vi "TLB Native Dynamic Events ver 0.26d.vi"() -> ()   [LabVIEW 2018] (continued)
          tunnel: w289 -> [_ _ _ _ _ _ _ _ _ _ _ _ _ _ _ _ _ _ _ _ _ _ _ _ _ _ _ _ _ _ _ _ _ _ _ _ _ _ _ _ _ _ _ _ _ _ _ _ _ _ _ _ _ _ _ _ _ _ _]
          tunnel: w288 -> [_ _ _ _ _ _ _ _ _ _ _ _ _ _ _ _ _ _ _ _ _ _ _ _ _ _ _ _ _ _ _ _ _ _ _ _ _ _ _ _ _ _ _ _ _ _ _ _ _ _ _ _ _ _ _ _ _ _ _]
          tunnel: w287 -> [_ _ _ _ _ _ _ _ _ _ _ _ _ _ _ _ _ _ _ _ _ _ _ _ _ _ _ _ _ _ _ _ _ _ _ _ _ _ _ _ _ _ w2183 _ w2271 _ _ _ _ _ _ _ _ _ _ w2774 _ _ _]
          frame 0 {
            # ">>> yStepper command>>>"
          }
          frame 1 {
            # ">>> yStepper command>>>"
            n215 = for {
              shift-right: [w366] -> w360
              shift-left: w363 -> [w365]
              tunnel: string[] ["INIT", "RESET ARM", "RESET FLAGS", "RESET YAW", "NAVX CALIBRATE"] -> [w364] mode=indexing
              n216 = Enqueue Element(queue=w365, element=w364) -> (queue out=w366:refnum<queue>)  [unwired: 2 in, 2 out]
            }
            n217 = Bundle By Name(cluster=w358, "yStepper desired"=u8 0) -> (w357:T20)
            n218 = Bundle By Name(cluster=w355, "ySpeed"=0.0, "xSpeed"=0.0, "wSpeed"=0.0) -> (w354:T19)
          }
          frame 3 {
            # ">>Action Queue>>"
            # ">>> Motor control cluster >>>"
            # ">>> yStepper command>>>"
            n219 = Flush Queue(queue=w373, error in (no error)=w372) -> ()  [unwired: 3 out]
            n220 = for {
              shift-right: [w379] -> w374
              shift-left: w375 -> [w378]
              tunnel: string[] ["STOP", "RESET ENCODERS", "RESET YAW", "RESET ARM", "RESET ALL SENSORS", "DISPOSE CAM BUFFERS", "DISPOSE PROC BUFFERS", "CAM CLOSE", ""] -> [w377] mode=indexing
              n221 = Enqueue Element(queue=w378, element=w377) -> (queue out=w379:refnum<queue>)  [unwired: 2 in, 2 out]
            }
          }
          frame 4, Default {
            # ">>> Motor control cluster >>>"
            # ">>> yStepper command>>>"
            n222 = Dequeue Element(queue=w391, timeout in ms (-1)=w390, error in (no error)=w386) -> (element=w389:T10)  [unwired: 3 out]
            n223 = case shown="\"Start Task 9\"" w389 {
              tunnel: [w394 w402 w410 w418 w426 w434 w442 w450 w458 w465 w475 w483 w490 w493] -> w385
              tunnel: w388 -> [w395 w403 w411 w419 w427 w435 w443 w451 w459 w466 w474 w482 w490 w494]
              tunnel: [State_Type_Definitions,_for_0.26g_versions_and_later_2."Task 1A" ("Enum") State_Type_Definitions,_for_0.26g_versions_and_later_2."Task 2:Raise Arm" ("Enum") State_Type_Definitions,_for_0.26g_versions_and_later_2."Task 3" ("Enum") State_Type_Definitions,_for_0.26g_versions_and_later_2."Task 4_A" ("Enum") State_Type_Definitions,_for_0.26g_versions_and_later_2."Task 5A" ("Enum") State_Type_Definitions,_for_0.26g_versions_and_later_2."Task 6_A" ("Enum") State_Type_Definitions,_for_0.26g_versions_and_later_2."Task 8A: RAISE ARM" ("Enum") State_Type_Definitions,_for_0.26g_versions_and_later_2."Task 8A: RAISE ARM" ("Enum") State_Type_Definitions,_for_0.26g_versions_and_later_2."Task 8A: RAISE ARM" ("Enum") State_Type_Definitions,_for_0.26g_versions_and_later_2."Task 8A: RAISE ARM" ("Enum") State_Type_Definitions,_for_0.26g_versions_and_later_2."Task 9A: Raise Arm" ("Enum") State_Type_Definitions,_for_0.26g_versions_and_later_2."Task A1: Task 9 Open cam" ("Enum") State_Type_Definitions,_for_0.26g_versions_and_later_2."Idle" ("Enum") State_Type_Definitions,_for_0.26g_versions_and_later_2."Shutdown" ("Enum")] -> w387
              tunnel: [enum16{"Ball", "Soap", "Gel", "Pipe", "None"}."None" ("Object recognition mode") enum16{"Ball", "Soap", "Gel", "Pipe", "None"}."None" ("Object recognition mode") enum16{"Ball", "Soap", "Gel", "Pipe", "None"}."None" ("Object recognition mode") enum16{"Ball", "Soap", "Gel", "Pipe", "None"}."None" ("Object recognition mode") enum16{"Ball", "Soap", "Gel", "Pipe", "None"}."None" ("Object recognition mode") enum16{"Ball", "Soap", "Gel", "Pipe", "None"}."None" ("Object recognition mode") enum16{"Ball", "Soap", "Gel", "Pipe", "None"}."Ball" ("Object recognition mode") enum16{"Ball", "Soap", "Gel", "Pipe", "None"}."Gel" ("Object recognition mode") enum16{"Ball", "Soap", "Gel", "Pipe", "None"}."Pipe" ("Object recognition mode") enum16{"Ball", "Soap", "Gel", "Pipe", "None"}."Soap" ("Object recognition mode") enum16{"Ball", "Soap", "Gel", "Pipe", "None"}."None" ("Object recognition mode") enum16{"Ball", "Soap", "Gel", "Pipe", "None"}."None" ("Object recognition mode") enum16{"Ball", "Soap", "Gel", "Pipe", "None"}."None" ("Object recognition mode") enum16{"Ball", "Soap", "Gel", "Pipe", "None"}."None" ("Object recognition mode")] -> w380
              frame "Start Task 1" {
                n224 = for {
                  shift-right: [w399] -> w394
                  shift-left: w395 -> [w398]
                  tunnel: string[] ["RESET ENCODERS", "RESET YAW", "FORWARD", "READ ENCODERS"] -> [w397] mode=indexing
                  n225 = Enqueue Element(queue=w398, element=w397) -> (queue out=w399:refnum<queue>)  [unwired: 2 in, 2 out]
                }
              }
              frame "Start Task 2" {
                n226 = for {
                  shift-right: [w407] -> w402
                  shift-left: w403 -> [w406]
                  tunnel: string[] ["RESET ENCODERS", "RESET YAW", "READ ULTRASONIC", "ARDUINO - ULTRASONIC"] -> [w405] mode=indexing
                  n227 = Enqueue Element(queue=w406, element=w405) -> (queue out=w407:refnum<queue>)  [unwired: 2 in, 2 out]
                }
              }
              frame "Start Task 3" {
                n228 = for {
                  shift-right: [w415] -> w410
                  shift-left: w411 -> [w414]
                  tunnel: string[] ["RESET ENCODERS", "READ ENCODERS", "R-ACW"] -> [w413] mode=indexing
                  n229 = Enqueue Element(queue=w414, element=w413) -> (queue out=w415:refnum<queue>)  [unwired: 2 in, 2 out]
                }
              }
              frame "Start Task 4" {
                n230 = for {
                  shift-right: [w423] -> w418
                  shift-left: w419 -> [w422]
                  tunnel: string[] ["RESET YAW", "RESET ENCODERS", "RESET ARM", "RESET FLAGS", "", ""] -> [w421] mode=indexing
                  n231 = Enqueue Element(queue=w422, element=w421) -> (queue out=w423:refnum<queue>)  [unwired: 2 in, 2 out]
                }
              }
              frame "Start Task 5" {
                n232 = for {
                  shift-right: [w431] -> w426
                  shift-left: w427 -> [w430]
                  tunnel: string[] ["RESET YAW", "RESET ENCODERS", "RESET ARM", "RESET ALL SENSORS", "", ""] -> [w429] mode=indexing
                  n233 = Enqueue Element(queue=w430, element=w429) -> (queue out=w431:refnum<queue>)  [unwired: 2 in, 2 out]
                }
              }
              frame "Start Task 6" {
                n234 = for {
                  shift-right: [w439] -> w434
                  shift-left: w435 -> [w438]
                  tunnel: string[] ["OPEN LOG CAM ", "", "", "", "", ""] -> [w437] mode=indexing
                  n235 = Enqueue Element(queue=w438, element=w437) -> (queue out=w439:refnum<queue>)  [unwired: 2 in, 2 out]
                }
              }
              frame "Start Task 8 - BALL" {
                n236 = for {
                  shift-right: [w447] -> w442
                  shift-left: w443 -> [w446]
                  tunnel: string[] ["RESET YAW", "RESET ENCODERS", "RESET ARM", "RESET FLAGS"] -> [w445] mode=indexing
                  n237 = Enqueue Element(queue=w446, element=w445) -> (queue out=w447:refnum<queue>)  [unwired: 2 in, 2 out]
                }
              }
              frame "Start Task 8 - Gel" {
                n238 = for {
                  shift-right: [w455] -> w450
                  shift-left: w451 -> [w454]
                  tunnel: string[] ["RESET YAW", "RESET ENCODERS", "RESET ARM", "RESET FLAGS"] -> [w453] mode=indexing
                  n239 = Enqueue Element(queue=w454, element=w453) -> (queue out=w455:refnum<queue>)  [unwired: 2 in, 2 out]
                }
              }
              frame "Start Task 8 - Pipe" {
                n240 = for {
                  shift-right: [w463] -> w458
                  shift-left: w459 -> [w462]
                  tunnel: string[] ["RESET YAW", "RESET ENCODERS", "RESET ARM", "RESET FLAGS"] -> [w461] mode=indexing
                  n241 = Enqueue Element(queue=w462, element=w461) -> (queue out=w463:refnum<queue>)  [unwired: 2 in, 2 out]
                }
              }
              frame "Start Task 8 - Soap" {
                n242 = for {
                  shift-right: [w471] -> w465
                  shift-left: w466 -> [w470]
                  tunnel: string[] ["RESET YAW", "RESET ENCODERS", "RESET ARM", "RESET FLAGS"] -> [w469] mode=indexing
                  n243 = Enqueue Element(queue=w470, element=w469) -> (queue out=w471:refnum<queue>)  [unwired: 2 in, 2 out]
                }
              }
              frame "Start Task 9" {
                n244 = for {
                  shift-right: [w479] -> w475
                  shift-left: w474 -> [w478]
                  tunnel: string[] ["Z STEPPER BOX HEIGHT", "READ STEPPER VALUES", "", ""] -> [w477] mode=indexing
                  n245 = Enqueue Element(queue=w478, element=w477) -> (queue out=w479:refnum<queue>)  [unwired: 2 in, 2 out]
                }
              }
              frame "Start Task A" {
                n246 = for {
                  shift-right: [w487] -> w483
                  shift-left: w482 -> [w486]
                  tunnel: string[] ["RESET ENCODERS", "READ ENCODERS", "RESET YAW", "Z STEPPER BOX HEIGHT"] -> [w485] mode=indexing
                  n247 = Enqueue Element(queue=w486, element=w485) -> (queue out=w487:refnum<queue>)  [unwired: 2 in, 2 out]
                }
              }
              frame "None", Default {
              }
              frame "Exit" {
                n248 = for {
                  shift-right: [w498] -> w493
                  shift-left: w494 -> [w497]
                  tunnel: string[] ["STOP", "RESET ENCODERS", "RESET YAW", "EXIT"] -> [w496] mode=indexing
                  n249 = Enqueue Element(queue=w497, element=w496) -> (queue out=w498:refnum<queue>)  [unwired: 2 in, 2 out]
                }
              }
            }
          }
          frame 5 {
            # ">> Item Selection Bias >>"
            # ">>> yStepper command>>>"
            n250 = for {
              shift-right: [w509] -> w503
              shift-left: w505 -> [w508]
              tunnel: string[] ["INIT", "RESET ENCODERS", "RESET FLAGS", "CAM CLOSE", "DISPOSE BUFFERS", "EXIT", ""] -> [w507] mode=indexing
              n251 = Enqueue Element(queue=w508, element=w507) -> (queue out=w509:refnum<queue>)  [unwired: 2 in, 2 out]
            }
          }
          frame 6 {
            # ">>> Motor control cluster >>>"
            # ">> Line detection >>"
            # ">> Checks if 1 metre moved >>"
            # ">>> yStepper command>>>"
            # "Use 250"
            n252 = Greater?(x=w519, y=265.0) -> (0:w513:bool)
            n253 = Dequeue Element(queue=w526, timeout in ms (-1)=w525, error in (no error)=w524) -> (element=w523:T10)  [unwired: 3 out]
            n254 = And(x=w512, y=w513) -> (x .and. y?=w510:bool)
            n255 = case shown="\"Start Task 1\", Default" w523 {
              tunnel: w511 -> [w527 _]
              tunnel: [w537 State_Type_Definitions,_for_0.26g_versions_and_later_2."True Stop" ("Enum")] -> w522
              tunnel: w521 -> [w535 w552]
              tunnel: [w534 w551] -> w520
              tunnel: [State_Type_Definitions,_for_0.26g_versions_and_later_2."Idle" ("Enum") State_Type_Definitions,_for_0.26g_versions_and_later_2."Shutdown" ("Enum")] -> w517
              tunnel: w510 -> [w528 _]
              frame "Start Task 1", Default {
                n256 = Or(x=w528, y=w527) -> (x .or. y?=w529:bool)
                n257 = case shown="True" w529 {
                  tunnel: w535 -> [w540 w546]
                  tunnel: [w539 w544] -> w534
                  frame False {
                    n258 = for {
                      shift-right: [w542] -> w539
                      shift-left: w540 -> [w543]
                      tunnel: string[] ["READ ENCODERS", "READ NAVX", "FORWARD", "READ LINE SENSOR"] ("element") -> [w541] mode=indexing
                      n259 = Enqueue Element(queue=w543, element=w541) -> (queue out=w542:refnum<queue>)  [unwired: 2 in, 2 out]
                    }
                  }
                  frame True {
                    n260 = for {
                      shift-right: [w548] -> w544
                      shift-left: w546 -> [w549]
                      tunnel: string[] ["RESET YAW", "RESET ENCODERS", "STOP", ""] -> [w547] mode=indexing
                      n261 = Enqueue Element(queue=w549, element=w547) -> (queue out=w548:refnum<queue>)  [unwired: 2 in, 2 out]
                    }
                  }
                }
                n262 = Select(t=State_Type_Definitions,_for_0.26g_versions_and_later_2."True Stop" ("Enum"), s=w527, f=State_Type_Definitions,_for_0.26g_versions_and_later_2."Task 1B" ("Enum")) -> (s? t:f=w532:T18)
                n263 = Select(t=w532, s=w528, f=State_Type_Definitions,_for_0.26g_versions_and_later_2."Task 1A" ("Enum")) -> (s? t:f=w537:T18)
              }
              frame "Exit" {
                n264 = for {
                  shift-right: [w556] -> w551
                  shift-left: w552 -> [w557]
                  tunnel: string[] ["STOP", "RESET ENCODERS", "RESET YAW", ""] -> [w555] mode=indexing
                  n265 = Enqueue Element(queue=w557, element=w555) -> (queue out=w556:refnum<queue>)  [unwired: 2 in, 2 out]
                }
              }
            }
          }
          frame 7 {
            # ">>> Motor control cluster >>>"
            # ">> Line detection >>"
            # ">> Adds small distance overhead after 1M >>"
            # ">>> yStepper command>>>"
            n266 = Greater?(x=w564, y=50.0) -> (0:w558:bool)
            n267 = Dequeue Element(queue=w573, timeout in ms (-1)=w572, error in (no error)=w571) -> (element=w570:T10)  [unwired: 3 out]
            n268 = Or(x=w558, y=w565) -> (x .or. y?=w569:bool)
            n269 = case shown="\"Start Task 1\", Default" w570 {
              tunnel: w569 -> [w576 _]
              tunnel: [w580 State_Type_Definitions,_for_0.26g_versions_and_later_2."True Stop" ("Enum")] -> w568
              tunnel: w567 -> [w577 w595]
              tunnel: [w575 w594] -> w566
              tunnel: [State_Type_Definitions,_for_0.26g_versions_and_later_2."Idle" ("Enum") State_Type_Definitions,_for_0.26g_versions_and_later_2."Shutdown" ("Enum")] -> w562
              frame "Start Task 1", Default {
                n270 = case shown="True" w576 {
                  tunnel: w577 -> [w583 w589]
                  tunnel: [w582 w587] -> w575
                  frame False {
                    n271 = for {
                      shift-right: [w585] -> w582
                      shift-left: w583 -> [w586]
                      tunnel: string[] ["READ ENCODERS", "READ NAVX", "FORWARD", "READ LINE SENSOR"] ("element") -> [w584] mode=indexing
                      n272 = Enqueue Element(queue=w586, element=w584) -> (queue out=w585:refnum<queue>)  [unwired: 2 in, 2 out]
                    }
                  }
                  frame True {
                    n273 = for {
                      shift-right: [w591] -> w587
                      shift-left: w589 -> [w592]
                      tunnel: string[] ["RESET YAW", "RESET ENCODERS", "STOP", ""] -> [w590] mode=indexing
                      n274 = Enqueue Element(queue=w592, element=w590) -> (queue out=w591:refnum<queue>)  [unwired: 2 in, 2 out]
                    }
                  }
                }
                n275 = Select(t=State_Type_Definitions,_for_0.26g_versions_and_later_2."True Stop" ("Enum"), s=w576, f=State_Type_Definitions,_for_0.26g_versions_and_later_2."Task 1B" ("Enum")) -> (s? t:f=w580:T18)
              }
              frame "Exit" {
                n276 = for {
                  shift-right: [w599] -> w594
                  shift-left: w595 -> [w600]
                  tunnel: string[] ["STOP", "RESET ENCODERS", "RESET YAW", ""] -> [w598] mode=indexing
                  n277 = Enqueue Element(queue=w600, element=w598) -> (queue out=w599:refnum<queue>)  [unwired: 2 in, 2 out]
                }
              }
            }
          }
          frame 8 {
            # ">> Stepper height reeached >>"
            # ">>> yStepper command>>>"
            # ">> Manual override >>"
            n278 = Dequeue Element(queue=w606, timeout in ms (-1)=w605, error in (no error)=w604) -> (element=w615:T10)  [unwired: 3 out]
            n279 = Equal?(x=w608, y=u8 60) -> (x = y?=w613:bool)
            n280 = case shown="\"Start Task 1\", Default" w615 {
              tunnel: [w626 State_Type_Definitions,_for_0.26g_versions_and_later_2."True Stop" ("Enum")] -> w610
              tunnel: [w624 w641] -> w603
              tunnel: w612 -> [w623 _]
              tunnel: w611 -> [w617 _]
              tunnel: [State_Type_Definitions,_for_0.26g_versions_and_later_2."Idle" ("Enum") State_Type_Definitions,_for_0.26g_versions_and_later_2."Shutdown" ("Enum")] -> w609
              tunnel: w613 -> [w616 _]
              frame "Start Task 1", Default {
                # ">> WIill proceed to part ii if not manual override >>"
                # ">>If ENABLE or Trigger is set to true>>"
                n281 = Or(x=w616, y=w617) -> (x .or. y?=w618:bool)
                n282 = case shown="True" w616 {
                  tunnel: [w629 w635] -> w624
                  tunnel: w623 -> [w628 w634]
                  frame False {
                    n283 = for {
                      shift-right: [w631] -> w629
                      shift-left: w628 -> [w632]
                      tunnel: string[] ["Z STEPPER CAM HEIGHT", "READ STEPPER VALUES"] ("element") -> [w630] mode=indexing
                      n284 = Enqueue Element(queue=w632, element=w630) -> (queue out=w631:refnum<queue>)  [unwired: 2 in, 2 out]
                    }
                  }
                  frame True {
                    n285 = for {
                      shift-right: [w637] -> w635
                      shift-left: w634 -> [w638]
                      tunnel: string[] ["ARDUINO - ULTRASONIC", "READ ULTRASONIC", "", "", "", ""] -> [w636] mode=indexing
                      n286 = Enqueue Element(queue=w638, element=w636) -> (queue out=w637:refnum<queue>)  [unwired: 2 in, 2 out]
                    }
                  }
                }
                n287 = Select(t=State_Type_Definitions,_for_0.26g_versions_and_later_2."True Stop" ("Enum"), s=w617, f=State_Type_Definitions,_for_0.26g_versions_and_later_2."Task 2:Sensor Mode" ("Enum")) -> (s? t:f=w620:T18)
                n288 = Select(t=w620, s=w618, f=State_Type_Definitions,_for_0.26g_versions_and_later_2."Task 2:Raise Arm" ("Enum")) -> (s? t:f=w626:T18)
              }
              frame "Exit" {
                n289 = for {
                  shift-right: [w644] -> w641
                  shift-left: _ -> [w645]
                  tunnel: string[] ["STOP", "RESET ENCODERS", "RESET YAW", ""] -> [w643] mode=indexing
                  n290 = Enqueue Element(queue=w645, element=w643) -> (queue out=w644:refnum<queue>)  [unwired: 2 in, 2 out]
                }
              }
            }
          }
          frame 9 {
            w662 = u8 20 ("y")
            # ">>> yStepper command>>>"
            # ">>Object detected>>"
            n291 = Dequeue Element(queue=w655, timeout in ms (-1)=w654, error in (no error)=w653) -> (element=w663:T10)  [unwired: 3 out]
            n292 = Less?(x=w651, y=w662) -> (x < y?=w661:bool)
            n293 = Less?(x=w650, y=w662) -> (x < y?=w660:bool)
            n294 = Or(x=w661, y=w660) -> (x .or. y?=w646:bool)
            n295 = case shown="\"Start Task 1\", Default" w663 {
              tunnel: w646 -> [w666 _]
              tunnel: [w673 State_Type_Definitions,_for_0.26g_versions_and_later_2."True Stop" ("Enum")] -> w659
              tunnel: w652 -> [w665 _]
              tunnel: w656 -> [w672 w689]
              tunnel: [w671 w690] -> w658
              tunnel: [State_Type_Definitions,_for_0.26g_versions_and_later_2."Idle" ("Enum") State_Type_Definitions,_for_0.26g_versions_and_later_2."Shutdown" ("Enum")] -> w657
              frame "Start Task 1", Default {
                n296 = case shown="False" w666 {
                  tunnel: w672 -> [w676 w683]
                  tunnel: [w677 w682] -> w671
                  frame False {
                    n297 = for {
                      tunnel: string[] ["READ ULTRASONIC", "STOP"] ("element") -> [w678] mode=indexing
                      shift-right: [w680] -> w677
                      shift-left: w676 -> [w679]
                      n298 = Enqueue Element(queue=w679, element=w678) -> (queue out=w680:refnum<queue>)  [unwired: 2 in, 2 out]
                    }
                  }
                  frame True {
                    n299 = for {
                      shift-right: [w685] -> w682
                      shift-left: w683 -> [w686]
                      tunnel: string[] ["RESET ENCODERS", "READ NAVX", "READ ENCODERS"] -> [w684] mode=indexing
                      n300 = Enqueue Element(queue=w686, element=w684) -> (queue out=w685:refnum<queue>)  [unwired: 2 in, 2 out]
                    }
                  }
                }
                n301 = Or(x=w666, y=w665) -> (x .or. y?=w664:bool)
                n302 = Select(t=State_Type_Definitions,_for_0.26g_versions_and_later_2."True Stop" ("Enum"), s=w665, f=State_Type_Definitions,_for_0.26g_versions_and_later_2."Task 2:Reverse Mode" ("Enum")) -> (s? t:f=w667:T18)
                n303 = Select(t=w667, s=w664, f=State_Type_Definitions,_for_0.26g_versions_and_later_2."Task 2:Sensor Mode" ("Enum")) -> (s? t:f=w673:T18)
              }
              frame "Exit" {
                n304 = for {
                  shift-right: [w693] -> w690
                  shift-left: w689 -> [w694]
                  tunnel: string[] ["STOP", "RESET ENCODERS", "RESET YAW", "ARDUINO MODE 0"] -> [w692] mode=indexing
                  n305 = Enqueue Element(queue=w694, element=w692) -> (queue out=w693:refnum<queue>)  [unwired: 2 in, 2 out]
                }
              }
            }
          }
          frame 10 {
            # ">>> yStepper command>>>"
            n306 = Dequeue Element(queue=w705, timeout in ms (-1)=w706, error in (no error)=w707) -> (element=w709:T10)  [unwired: 3 out]
            n307 = Less?(x=w699, y=-50.0) -> (x < y?=w697:bool)
            n308 = case shown="\"Start Task 1\", Default" w709 {
              tunnel: [w719 State_Type_Definitions,_for_0.26g_versions_and_later_2."True Stop" ("Enum")] -> w701
              tunnel: w708 -> [w712 _]
              tunnel: w704 -> [w718 w735]
              tunnel: [w717 w736] -> w700
              tunnel: [State_Type_Definitions,_for_0.26g_versions_and_later_2."Idle" ("Enum") State_Type_Definitions,_for_0.26g_versions_and_later_2."Shutdown" ("Enum")] -> w702
              tunnel: w697 -> [w710 _]
              frame "Start Task 1", Default {
                n309 = case shown="True" w710 {
                  tunnel: w718 -> [w722 w729]
                  tunnel: [w723 w728] -> w717
                  frame False {
                    n310 = for {
                      tunnel: string[] ["READ ENCODERS", "REVERSE", "READ NAVX"] ("element") -> [w724] mode=indexing
                      shift-right: [w726] -> w723
                      shift-left: w722 -> [w725]
                      n311 = Enqueue Element(queue=w725, element=w724) -> (queue out=w726:refnum<queue>)  [unwired: 2 in, 2 out]
                    }
                  }
                  frame True {
                    n312 = for {
                      shift-right: [w731] -> w728
                      shift-left: w729 -> [w732]
                      tunnel: string[] ["STOP", "ARDUINO - ULTRASONIC", "READ ULTRASONIC", "RESET ENCODERS"] -> [w730] mode=indexing
                      n313 = Enqueue Element(queue=w732, element=w730) -> (queue out=w731:refnum<queue>)  [unwired: 2 in, 2 out]
                    }
                  }
                }
                n314 = Or(x=w710, y=w712) -> (x .or. y?=w711:bool)
                n315 = Select(t=State_Type_Definitions,_for_0.26g_versions_and_later_2."True Stop" ("Enum"), s=w712, f=State_Type_Definitions,_for_0.26g_versions_and_later_2."Task 2:Sensor Mode" ("Enum")) -> (s? t:f=w713:T18)
                n316 = Select(t=w713, s=w711, f=State_Type_Definitions,_for_0.26g_versions_and_later_2."Task 2:Reverse Mode" ("Enum")) -> (s? t:f=w719:T18)
              }
              frame "Exit" {
                n317 = for {
                  shift-right: [w739] -> w736
                  shift-left: w735 -> [w740]
                  tunnel: string[] ["STOP", "RESET ENCODERS", "RESET YAW", "ARDUINO MODE 0"] -> [w738] mode=indexing
                  n318 = Enqueue Element(queue=w740, element=w738) -> (queue out=w739:refnum<queue>)  [unwired: 2 in, 2 out]
                }
              }
            }
          }
          frame 11 {
            # ">>> Motor control cluster >>>"
            # ">>> yStepper command>>>"
            n319 = Dequeue Element(queue=w756, timeout in ms (-1)=w755, error in (no error)=w754) -> (element=w745:T10)  [unwired: 3 out]
            n320 = Less?(x=w753, y=-160.0) -> (x < y?=w750:bool)
            n321 = Or(x=w750, y=w751) -> (x .or. y?=w746:bool)
            n322 = case shown="\"Start Task 1\", Default" w745 {
              tunnel: w746 -> [w759 _]
              tunnel: [w763 State_Type_Definitions,_for_0.26g_versions_and_later_2."True Stop" ("Enum")] -> w747
              tunnel: w749 -> [w760 w779]
              tunnel: [w758 w778] -> w748
              tunnel: [State_Type_Definitions,_for_0.26g_versions_and_later_2."Idle" ("Enum") State_Type_Definitions,_for_0.26g_versions_and_later_2."Shutdown" ("Enum")] -> w744
              frame "Start Task 1", Default {
                n323 = case shown="False" w759 {
                  tunnel: w760 -> [w766 w772]
                  tunnel: [w765 w770] -> w758
                  frame False {
                    n324 = for {
                      shift-right: [w768] -> w765
                      shift-left: w766 -> [w769]
                      tunnel: string[] ["READ ENCODERS", "R-CW"] ("element") -> [w767] mode=indexing
                      n325 = Enqueue Element(queue=w769, element=w767) -> (queue out=w768:refnum<queue>)  [unwired: 2 in, 2 out]
                    }
                  }
                  frame True {
                    n326 = for {
                      shift-right: [w774] -> w770
                      shift-left: w772 -> [w775]
                      tunnel: string[] ["RESET YAW", "RESET ENCODERS", "STOP", "ARDUINO MODE 0"] -> [w773] mode=indexing
                      n327 = Enqueue Element(queue=w775, element=w773) -> (queue out=w774:refnum<queue>)  [unwired: 2 in, 2 out]
                    }
                  }
                }
                n328 = Select(t=State_Type_Definitions,_for_0.26g_versions_and_later_2."True Stop" ("Enum"), s=w759, f=State_Type_Definitions,_for_0.26g_versions_and_later_2."Task 3" ("Enum")) -> (s? t:f=w763:T18)
              }
              frame "Exit" {
                n329 = for {
                  shift-right: [w782] -> w778
                  shift-left: w779 -> [w783]
                  tunnel: string[] ["STOP", "RESET ENCODERS", "RESET YAW", ""] -> [w781] mode=indexing
                  n330 = Enqueue Element(queue=w783, element=w781) -> (queue out=w782:refnum<queue>)  [unwired: 2 in, 2 out]
                }
              }
            }
          }
          frame 12 {
            # ">> Stepper height reeached >>"
            # ">>> yStepper command>>>"
            # ">> Manual override >>"
            n331 = Dequeue Element(queue=w797, timeout in ms (-1)=w796, error in (no error)=w795) -> (element=w794:T10)  [unwired: 3 out]
            n332 = Equal?(x=w788, y=u8 60) -> (x = y?=w786:bool)
            n333 = case shown="\"Start Task 1\", Default" w794 {
              tunnel: [w809 State_Type_Definitions,_for_0.26g_versions_and_later_2."True Stop" ("Enum")] -> w793
              tunnel: [w807 w825] -> w792
              tunnel: w798 -> [w806 w822]
              tunnel: w791 -> [w800 _]
              tunnel: [State_Type_Definitions,_for_0.26g_versions_and_later_2."Idle" ("Enum") State_Type_Definitions,_for_0.26g_versions_and_later_2."Shutdown" ("Enum")] -> w790
              tunnel: w786 -> [w799 _]
              frame "Start Task 1", Default {
                # ">> WIill proceed to part ii if not manual override >>"
                # ">>If ENABLE or Trigger is set to true>>"
                n334 = Or(x=w799, y=w800) -> (x .or. y?=w801:bool)
                n335 = case shown="False" w799 {
                  tunnel: [w812 w818] -> w807
                  tunnel: w806 -> [w811 w817]
                  frame False {
                    n336 = for {
                      shift-right: [w814] -> w812
                      shift-left: w811 -> [w815]
                      tunnel: string[] ["Z STEPPER CAM HEIGHT", "READ STEPPER VALUES"] ("element") -> [w813] mode=indexing
                      n337 = Enqueue Element(queue=w815, element=w813) -> (queue out=w814:refnum<queue>)  [unwired: 2 in, 2 out]
                    }
                  }
                  frame True {
                    n338 = for {
                      shift-right: [w820] -> w818
                      shift-left: w817 -> [w821]
                      tunnel: string[] ["ARDUINO - ULTRASONIC", "READ ULTRASONIC", "FORWARD", "", "", ""] -> [w819] mode=indexing
                      n339 = Enqueue Element(queue=w821, element=w819) -> (queue out=w820:refnum<queue>)  [unwired: 2 in, 2 out]
                    }
                  }
                }
                n340 = Select(t=State_Type_Definitions,_for_0.26g_versions_and_later_2."True Stop" ("Enum"), s=w800, f=State_Type_Definitions,_for_0.26g_versions_and_later_2."Task 4_B" ("Enum")) -> (s? t:f=w803:T18)
                n341 = Select(t=w803, s=w801, f=State_Type_Definitions,_for_0.26g_versions_and_later_2."Task 4_A" ("Enum")) -> (s? t:f=w809:T18)
              }
              frame "Exit" {
                n342 = for {
                  shift-right: [w828] -> w825
                  shift-left: w822 -> [w829]
                  tunnel: string[] ["STOP", "RESET ENCODERS", "RESET YAW", ""] -> [w827] mode=indexing
                  n343 = Enqueue Element(queue=w829, element=w827) -> (queue out=w828:refnum<queue>)  [unwired: 2 in, 2 out]
                }
              }
            }
          }
          frame 13 {
            w835 = u8 20
            # ">> Path blocked >>"
            # ">>> yStepper command>>>"
            # ">> Manual override >>"
            n344 = Dequeue Element(queue=w844, timeout in ms (-1)=w843, error in (no error)=w842) -> (element=w841:T10)  [unwired: 3 out]
            n345 = Less?(x=w837, y=w835) -> (x < y?=w832:bool)
            n346 = Less?(x=w836, y=w835) -> (x < y?=w833:bool)
            n347 = And(x=w833, y=w832) -> (x .and. y?=w834:bool)
            n348 = case shown="\"Start Task 1\", Default" w841 {
              tunnel: [w858 State_Type_Definitions,_for_0.26g_versions_and_later_2."True Stop" ("Enum")] -> w846
              tunnel: [w856 w873] -> w847
              tunnel: w840 -> [w855 _]
              tunnel: w845 -> [w849 _]
              tunnel: [State_Type_Definitions,_for_0.26g_versions_and_later_2."Idle" ("Enum") State_Type_Definitions,_for_0.26g_versions_and_later_2."Shutdown" ("Enum")] -> w839
              tunnel: w834 -> [w848 _]
              frame "Start Task 1", Default {
                # ">> Manual override forces program to true stop >>"
                # ">>If ENABLE or Trigger is set to true>>"
                n349 = Or(x=w848, y=w849) -> (x .or. y?=w854:bool)
                n350 = case shown="False" w848 {
                  tunnel: [w861 w866] -> w856
                  tunnel: w855 -> [w860 w865]
                  frame False {
                    n351 = for {
                      shift-right: [w863] -> w861
                      shift-left: w860 -> [w864]
                      tunnel: string[] ["FORWARD", "READ ULTRASONIC", "READ NAVX"] ("element") -> [w862] mode=indexing
                      n352 = Enqueue Element(queue=w864, element=w862) -> (queue out=w863:refnum<queue>)  [unwired: 2 in, 2 out]
                    }
                  }
                  frame True {
                    n353 = for {
                      shift-right: [w869] -> w866
                      shift-left: w865 -> [w870]
                      tunnel: string[] ["STOP", "RESET YAW", "RESET ENCODERS", "RESET FLAGS"] -> [w868] mode=indexing
                      n354 = Enqueue Element(queue=w870, element=w868) -> (queue out=w869:refnum<queue>)  [unwired: 2 in, 2 out]
                    }
                  }
                }
                n355 = Select(t=State_Type_Definitions,_for_0.26g_versions_and_later_2."True Stop" ("Enum"), s=w849, f=State_Type_Definitions,_for_0.26g_versions_and_later_2."Task 4_C" ("Enum")) -> (s? t:f=w851:T18)
                n356 = Select(t=w851, s=w854, f=State_Type_Definitions,_for_0.26g_versions_and_later_2."Task 4_B" ("Enum")) -> (s? t:f=w858:T18)
              }
              frame "Exit" {
                n357 = for {
                  shift-right: [w876] -> w873
                  shift-left: _ -> [w877]
                  tunnel: string[] ["STOP", "RESET ENCODERS", "RESET YAW", ""] -> [w875] mode=indexing
                  n358 = Enqueue Element(queue=w877, element=w875) -> (queue out=w876:refnum<queue>)  [unwired: 2 in, 2 out]
                }
              }
            }
          }
          frame 14 {
            w889 = u8 20
            # ">> xDistance travelled>>"
            # ">> Path NOT blocked >>"
            # ">>> yStepper command>>>"
            # ">> Manual override >>"
            n359 = Dequeue Element(queue=w899, timeout in ms (-1)=w892, error in (no error)=w891) -> (element=w893:T10)  [unwired: 3 out]
            n360 = Greater?(x=w881, y=w889) -> (0:w887:bool)
            n361 = Greater?(x=w886, y=80.0) -> (0:w884:bool)
            n362 = Greater?(x=w880, y=w889) -> (0:w888:bool)
            n363 = And(x=w888, y=w887) -> (x .and. y?=w883:bool)
            n364 = And(x=w884, y=w883) -> (x .and. y?=w882:bool)
            n365 = case shown="\"Start Task 1\", Default" w893 {
              tunnel: [w910 State_Type_Definitions,_for_0.26g_versions_and_later_2."True Stop" ("Enum")] -> w896
              tunnel: [w908 w926] -> w895
              tunnel: w898 -> [w907 w923]
              tunnel: w897 -> [w901 _]
              tunnel: [State_Type_Definitions,_for_0.26g_versions_and_later_2."Idle" ("t") State_Type_Definitions,_for_0.26g_versions_and_later_2."Shutdown" ("Enum")] -> w894
              tunnel: w882 -> [w900 _]
              frame "Start Task 1", Default {
                # ">> Manual override forces program to true stop >>"
                # ">>If ENABLE or Trigger is set to true>>"
                n366 = Or(x=w900, y=w901) -> (x .or. y?=w906:bool)
                n367 = case shown="False" w900 {
                  tunnel: [w913 w918] -> w908
                  tunnel: w907 -> [w911 w917]
                  frame False {
                    n368 = for {
                      shift-right: [w915] -> w913
                      shift-left: w911 -> [w916]
                      tunnel: string[] ["RIGHT", "READ NAVX", "READ ENCODERS", "READ ULTRASONIC"] ("element") -> [w914] mode=indexing
                      n369 = Enqueue Element(queue=w916, element=w914) -> (queue out=w915:refnum<queue>)  [unwired: 2 in, 2 out]
                    }
                  }
                  frame True {
                    n370 = for {
                      shift-right: [w921] -> w918
                      shift-left: w917 -> [w922]
                      tunnel: string[] ["STOP", "RESET YAW", "RESET ENCODERS", "ARDUINO - ULTRASONIC"] -> [w920] mode=indexing
                      n371 = Enqueue Element(queue=w922, element=w920) -> (queue out=w921:refnum<queue>)  [unwired: 2 in, 2 out]
                    }
                  }
                }
                n372 = Select(t=State_Type_Definitions,_for_0.26g_versions_and_later_2."True Stop" ("Enum"), s=w901, f=State_Type_Definitions,_for_0.26g_versions_and_later_2."Task 4_D" ("Enum")) -> (s? t:f=w902:T18)
                n373 = Select(t=w902, s=w906, f=State_Type_Definitions,_for_0.26g_versions_and_later_2."Task 4_C" ("Enum")) -> (s? t:f=w910:T18)
              }
              frame "Exit" {
                n374 = for {
                  shift-right: [w929] -> w926
                  shift-left: w923 -> [w930]
                  tunnel: string[] ["STOP", "RESET ENCODERS", "RESET YAW", ""] -> [w928] mode=indexing
                  n375 = Enqueue Element(queue=w930, element=w928) -> (queue out=w929:refnum<queue>)  [unwired: 2 in, 2 out]
                }
              }
            }
          }
          frame 15 {
            w953 = u8 20
            # ">>> Motor control cluster >>>"
            # ">> Line detected >>"
            # ">> yDistance travelled>>"
            # ">> Path blocked >>"
            # ">>> yStepper command>>>"
            # ">> Manual override >>"
            n376 = Less?(x=w938, y=w953) -> (x < y?=w951:bool)
            n377 = Greater?(x=w942, y=200.0) -> (0:w949:bool)
            n378 = Less?(x=w937, y=w953) -> (x < y?=w952:bool)
            n379 = And(x=w952, y=w951) -> (x .and. y?=w948:bool)
            n380 = Dequeue Element(queue=w945, timeout in ms (-1)=w944, error in (no error)=w943) -> (element=w954:T10)  [unwired: 3 out]
            n381 = Or(x=w949, y=w948) -> (x .or. y?=w932:bool)
            n382 = And(x=w933, y=w932) -> (x .and. y?=w931:bool)
            n383 = case shown="\"Start Task 1\", Default" w954 {
              tunnel: [w965 State_Type_Definitions,_for_0.26g_versions_and_later_2."True Stop" ("Enum")] -> w941
              tunnel: [w963 w981] -> w939
              tunnel: w946 -> [w962 w978]
              tunnel: w947 -> [w956 _]
              tunnel: [State_Type_Definitions,_for_0.26g_versions_and_later_2."Idle" ("t") State_Type_Definitions,_for_0.26g_versions_and_later_2."Shutdown" ("Enum")] -> w940
              tunnel: w931 -> [w955 _]
              frame "Start Task 1", Default {
                # ">> Manual override forces program to true stop >>"
                # ">>If ENABLE or Trigger is set to true>>"
                n384 = Or(x=w955, y=w956) -> (x .or. y?=w961:bool)
                n385 = case shown="False" w955 {
                  tunnel: [w968 w973] -> w963
                  tunnel: w962 -> [w966 w972]
                  frame False {
                    n386 = for {
                      shift-right: [w970] -> w968
                      shift-left: w966 -> [w971]
                      tunnel: string[] ["FORWARD", "READ NAVX", "READ ENCODERS", "READ ULTRASONIC", "READ LINE SENSOR"] ("element") -> [w969] mode=indexing
                      n387 = Enqueue Element(queue=w971, element=w969) -> (queue out=w970:refnum<queue>)  [unwired: 2 in, 2 out]
                    }
                  }
                  frame True {
                    n388 = for {
                      shift-right: [w976] -> w973
                      shift-left: w972 -> [w977]
                      tunnel: string[] ["STOP", "RESET YAW", "RESET ENCODERS", "RESET FLAGS"] -> [w975] mode=indexing
                      n389 = Enqueue Element(queue=w977, element=w975) -> (queue out=w976:refnum<queue>)  [unwired: 2 in, 2 out]
                    }
                  }
                }
                n390 = Select(t=State_Type_Definitions,_for_0.26g_versions_and_later_2."True Stop" ("Enum"), s=w956, f=State_Type_Definitions,_for_0.26g_versions_and_later_2."True Stop" ("Enum")) -> (s? t:f=w957:T18)
                n391 = Select(t=w957, s=w961, f=State_Type_Definitions,_for_0.26g_versions_and_later_2."Task 4_D" ("Enum")) -> (s? t:f=w965:T18)
              }
              frame "Exit" {
                n392 = for {
                  shift-right: [w984] -> w981
                  shift-left: w978 -> [w985]
                  tunnel: string[] ["STOP", "RESET ENCODERS", "RESET YAW", ""] -> [w983] mode=indexing
                  n393 = Enqueue Element(queue=w985, element=w983) -> (queue out=w984:refnum<queue>)  [unwired: 2 in, 2 out]
                }
              }
            }
          }
          frame 16 {
            # "Stays in Task 5_A until stepper reaches desired \nheight"
            # ">>> Motor control cluster >>>"
            # ">>> yStepper command>>>"
            # ">> Manual override >>"
            n394 = Dequeue Element(queue=w996, timeout in ms (-1)=w995, error in (no error)=w997) -> (element=w994:T10)  [unwired: 3 out]
            n395 = Equal?(x=w993, y=u8 1) -> (x = y?=w991:bool)
            n396 = case shown="\"Start Task 1\", Default" w994 {
              tunnel: [w1007 State_Type_Definitions,_for_0.26g_versions_and_later_2."True Stop" ("Enum")] -> w998
              tunnel: [w1010 w1027] -> w999
              tunnel: [State_Type_Definitions,_for_0.26g_versions_and_later_2."Idle" ("Enum") State_Type_Definitions,_for_0.26g_versions_and_later_2."Shutdown" ("Enum")] -> w1000
              tunnel: w991 -> [w1006 _]
              tunnel: w990 -> [w1005 _]
              tunnel: w989 -> [w1001 w1024]
              frame "Start Task 1", Default {
                # "T: Go back to idle, F: Continue with task\""
                # ">> Manual override >>"
                n397 = case shown="True" w1006 {
                  tunnel: [w1014 w1020] -> w1010
                  tunnel: w1001 -> [w1012 w1018]
                  frame False {
                    n398 = for {
                      tunnel: string[] ["Z STEPPER GRAB HEIGHT", "READ STEPPER VALUES"] ("element") -> [w1015] mode=indexing
                      shift-right: [w1017] -> w1014
                      shift-left: w1012 -> [w1016]
                      n399 = Enqueue Element(queue=w1016, element=w1015) -> (queue out=w1017:refnum<queue>)  [unwired: 2 in, 2 out]
                    }
                  }
                  frame True {
                    n400 = for {
                      shift-right: [w1022] -> w1020
                      shift-left: w1018 -> [w1023]
                      tunnel: string[] ["SET TIMER 2", "", ""] -> [w1021] mode=indexing
                      n401 = Enqueue Element(queue=w1023, element=w1021) -> (queue out=w1022:refnum<queue>)  [unwired: 2 in, 2 out]
                    }
                  }
                }
                n402 = Or(x=w1006, y=w1005) -> (x .or. y?=w1008:bool)
                n403 = Select(t=State_Type_Definitions,_for_0.26g_versions_and_later_2."True Stop" ("Enum"), s=w1005, f=State_Type_Definitions,_for_0.26g_versions_and_later_2."Task 5B" ("Enum")) -> (s? t:f=w1002:T18)
                n404 = Select(t=w1002, s=w1008, f=State_Type_Definitions,_for_0.26g_versions_and_later_2."Task 5A" ("Enum")) -> (s? t:f=w1007:T18)
              }
              frame "Exit" {
                n405 = for {
                  shift-right: [w1030] -> w1027
                  shift-left: w1024 -> [w1031]
                  tunnel: string[] ["STOP", "RESET ENCODERS", "RESET YAW", "ARDUINO MODE 0"] -> [w1029] mode=indexing
                  n406 = Enqueue Element(queue=w1031, element=w1029) -> (queue out=w1030:refnum<queue>)  [unwired: 2 in, 2 out]
                }
              }
            }
          }
          frame 17 {
            # ">>> yStepper command>>>"
            n407 = Dequeue Element(queue=w1038, timeout in ms (-1)=w1037, error in (no error)=w1039) -> (element=w1036:T10)  [unwired: 3 out]
            n408 = case shown="\"Start Task 1\", Default" w1036 {
              tunnel: [w1051 State_Type_Definitions,_for_0.26g_versions_and_later_2."True Stop" ("Enum")] -> w1041
              tunnel: [w1054 w1071] -> w1040
              tunnel: [State_Type_Definitions,_for_0.26g_versions_and_later_2."Idle" ("Enum") State_Type_Definitions,_for_0.26g_versions_and_later_2."Shutdown" ("Enum")] -> w1042
              tunnel: w1044 -> [w1050 _]
              tunnel: w1043 -> [w1046 w1068]
              tunnel: w1032 -> [w1045 _]
              frame "Start Task 1", Default {
                # "T: Go back to idle, F: Continue with task\""
                # ">> Manual override >>"
                n409 = case shown="True" w1045 {
                  tunnel: [w1058 w1064] -> w1054
                  tunnel: w1046 -> [w1056 w1062]
                  frame False {
                    n410 = for {
                      tunnel: string[] ["CLOSE CLAW", "START TIMER", ""] ("element") -> [w1059] mode=indexing
                      shift-right: [w1061] -> w1058
                      shift-left: w1056 -> [w1060]
                      n411 = Enqueue Element(queue=w1060, element=w1059) -> (queue out=w1061:refnum<queue>)  [unwired: 2 in, 2 out]
                    }
                  }
                  frame True {
                    n412 = for {
                      shift-right: [w1066] -> w1064
                      shift-left: w1062 -> [w1067]
                      tunnel: string[] ["STOP", "", "", ""] -> [w1065] mode=indexing
                      n413 = Enqueue Element(queue=w1067, element=w1065) -> (queue out=w1066:refnum<queue>)  [unwired: 2 in, 2 out]
                    }
                  }
                }
                n414 = Or(x=w1045, y=w1050) -> (x .or. y?=w1052:bool)
                n415 = Select(t=State_Type_Definitions,_for_0.26g_versions_and_later_2."True Stop" ("Enum"), s=w1050, f=State_Type_Definitions,_for_0.26g_versions_and_later_2."Task 5C" ("Enum")) -> (s? t:f=w1047:T18)
                n416 = Select(t=w1047, s=w1052, f=State_Type_Definitions,_for_0.26g_versions_and_later_2."Task 5B" ("Enum")) -> (s? t:f=w1051:T18)
              }
              frame "Exit" {
                n417 = for {
                  shift-right: [w1074] -> w1071
                  shift-left: w1068 -> [w1075]
                  tunnel: string[] ["STOP", "RESET ENCODERS", "RESET YAW", "ARDUINO MODE 0"] -> [w1073] mode=indexing
                  n418 = Enqueue Element(queue=w1075, element=w1073) -> (queue out=w1074:refnum<queue>)  [unwired: 2 in, 2 out]
                }
              }
            }
          }
          frame 18 {
            # ">>> Motor control cluster >>>"
            # ">>> yStepper command>>>"
            # ">> Manual override >>"
            n419 = Equal?(x=w1078, y=u8 60) -> (x = y?=w1076:bool)
            n420 = Dequeue Element(queue=w1088, timeout in ms (-1)=w1087, error in (no error)=w1086) -> (element=w1085:T10)  [unwired: 3 out]
            n421 = case shown="\"Start Task 1\", Default" w1085 {
              tunnel: [w1097 State_Type_Definitions,_for_0.26g_versions_and_later_2."True Stop" ("Enum")] -> w1090
              tunnel: [w1100 w1117] -> w1083
              tunnel: [State_Type_Definitions,_for_0.26g_versions_and_later_2."Idle" ("Enum") State_Type_Definitions,_for_0.26g_versions_and_later_2."Shutdown" ("Enum")] -> w1082
              tunnel: w1084 -> [w1091 _]
              tunnel: w1089 -> [w1096 w1114]
              tunnel: w1076 -> [w1095 _]
              frame "Start Task 1", Default {
                # ">> Is time up? >>"
                # "Determines if object is in range to pick up"
                # ">> Manual override >>"
                n422 = case shown="True" w1095 {
                  tunnel: [w1104 w1110] -> w1100
                  tunnel: w1096 -> [w1102 w1108]
                  frame False {
                    n423 = for {
                      tunnel: string[] ["Z STEPPER CAM HEIGHT", "READ STEPPER VALUES"] ("element") -> [w1105] mode=indexing
                      shift-right: [w1107] -> w1104
                      shift-left: w1102 -> [w1106]
                      n424 = Enqueue Element(queue=w1106, element=w1105) -> (queue out=w1107:refnum<queue>)  [unwired: 2 in, 2 out]
                    }
                  }
                  frame True {
                    n425 = for {
                      shift-right: [w1112] -> w1110
                      shift-left: w1108 -> [w1113]
                      tunnel: string[] ["SET TIMER 5", "", ""] -> [w1111] mode=indexing
                      n426 = Enqueue Element(queue=w1113, element=w1111) -> (queue out=w1112:refnum<queue>)  [unwired: 2 in, 2 out]
                    }
                  }
                }
                n427 = Or(x=w1095, y=w1091) -> (x .or. y?=w1098:bool)
                n428 = Select(t=State_Type_Definitions,_for_0.26g_versions_and_later_2."True Stop" ("Enum"), s=w1091, f=State_Type_Definitions,_for_0.26g_versions_and_later_2."Task 5D" ("Enum")) -> (s? t:f=w1093:T18)
                n429 = Select(t=w1093, s=w1098, f=State_Type_Definitions,_for_0.26g_versions_and_later_2."Task 5C" ("Enum")) -> (s? t:f=w1097:T18)
              }
              frame "Exit" {
                n430 = for {
                  shift-right: [w1120] -> w1117
                  shift-left: w1114 -> [w1121]
                  tunnel: string[] ["STOP", "RESET ENCODERS", "RESET YAW", "ARDUINO MODE 0"] -> [w1119] mode=indexing
                  n431 = Enqueue Element(queue=w1121, element=w1119) -> (queue out=w1120:refnum<queue>)  [unwired: 2 in, 2 out]
                }
              }
            }
          }
          frame 19 {
            # ">>> yStepper command>>>"
            n432 = Dequeue Element(queue=w1129, timeout in ms (-1)=w1128, error in (no error)=w1127) -> (element=w1126:T10)  [unwired: 3 out]
            n433 = case shown="\"Start Task 1\", Default" w1126 {
              tunnel: [w1141 State_Type_Definitions,_for_0.26g_versions_and_later_2."True Stop" ("Enum")] -> w1133
              tunnel: [w1144 w1161] -> w1132
              tunnel: [State_Type_Definitions,_for_0.26g_versions_and_later_2."Idle" ("Enum") State_Type_Definitions,_for_0.26g_versions_and_later_2."Shutdown" ("Enum")] -> w1134
              tunnel: w1130 -> [w1140 _]
              tunnel: w1131 -> [w1136 w1158]
              tunnel: w1124 -> [w1135 _]
              frame "Start Task 1", Default {
                # ">> T: Breaks out of state loop; F: Stays in loop>>"
                # ">> Manual override >>"
                # ">> Checks if time is up>>"
                # "Stays in Task 5D until the object is detected"
                # "T: Go back to idle, F: Continue with task\""
                # ">> Manual override >>"
                n434 = case shown="False" w1135 {
                  tunnel: [w1148 w1154] -> w1144
                  tunnel: w1136 -> [w1146 w1152]
                  frame False {